vi "pharmaBot_v0.019.vi"() -> ()   [LabVIEW 2015]
uses:
  controls/user_message_v6.ctl
  pipette cleaning/pressure box/cleaning_soft/controls/arduino_pressure_setting.ctl
  <vilib>/vision/NI_Vision_Development_Module.lvlib
  <vilib>/vision/Image Controls.llb/IMAQ Image.ctl
  multiBot/patcherBot/AxMultiClampMsg.dll
  <vilib>/Platform/NI_3dgraph.lvlib
  controls/cam_type-v02.ctl
  controls/cam_info.ctl
  machine_vision/controls/transform_cluster_actuator.ctl
  <vilib>/Analysis/NI_AALBLAS.lvlib
  <vilib>/Analysis/BLAS.llb/dnrm2 - Vector 2-Norm (DBL).vi
  multipatch/controls/multipatch_individual_controls_v5.ctl
  multipatch/controls/images_controls.ctl
  machine_vision/controls/approach_type.ctl
  controls/scope_motion.ctl
  <vilib>/ptbypt/NI_PtbyPt.lvlib
  pipette cleaning/pressure box/cleaning_soft/controls/scientifica_commands.ctl
  multipatch/controls/multipatch_common_controls_v4.ctl
  controls/Load and Save Controls_LV2009.llb/RWC_Actions.ctl
  controls/memtest_def.ctl
  pipette cleaning/pressure box/cleaning_soft/controls/actuator_type.ctl
  pipette cleaning/pressure box/cleaning_soft/controls/actuator_cluster.ctl
  pipette cleaning/pressure box/cleaning_soft/controls/pressure_box_type.ctl
  pipette cleaning/pressure box/cleaning_soft/controls/pressure_box_control.ctl
  machine_vision/coordinate model vis/transform_properties_actuators.ctl
  controls/NH_method.ctl
  controls/dual_patch_controls.ctl
  wc_protocol_v1.003 Folder/whole_cell_protocol/Controls/cell_stats-v02.ctl
  multipatch/controls/Control 7b.ctl
  controls/notSureControl-v01.ctl
panel:
  in  "misc indiv":T1
  in  "Save Resistance":bool
  out "Saved Pipette Resistance":dbl caption="MOhms" format="%#_3g"
  out "allMainVIcontrols":refnum<vi>[](array[refnum])
  out "cells selected":i32
  in  "unpatched+reserved 2":i32[](array[numeric])
  out "cells left":i32
  out "ValidationOutputCluster":T2(array[cluster])=[{"daq_ao 2"="Dev1/ao1", "Duration (s)"=10.0, "Sample Freq (Hz)"=20000.0, "Phase"=-36.0, "Duty Cycle"=10.0, "Jump Filter Freq (Hz)"=30.0, "Number of Replicates"=1}, {"daq_ao 2"="", "Duration (s)"=0.0, "Sample Freq (Hz)"=0.0, "Phase"=0.0, "Duty Cycle"=0.0, "Jump Filter Freq (Hz)"=0.0, "Number of Replicates"=0}, {"daq_ao 2"="Dev1/ao1", "Duration (s)"=10.0, "Sample Freq (Hz)"=20000.0, "Phase"=-36.0, "Duty Cycle"=10.0, "Jump Filter Freq (Hz)"=30.0, "Number of Replicates"=1}, {"daq_ao 2"="Dev1/ao1", "Duration (s)"=10.0, "Sample Freq (Hz)"=20000.0, "Phase"=-36.0, "Duty Cycle"=10.0, "Jump Filter Freq (Hz)"=30.0, "Number of Replicates"=1}, {"daq_ao 2"="Dev1/ao1", "Duration (s)"=10.0, "Sample Freq (Hz)"=20000.0, "Phase"=-36.0, "Duty Cycle"=10.0, "Jump Filter Freq (Hz)"=30.0, "Number of Replicates"=1}, {"daq_ao 2"="", "Duration (s)"=0.0, "Sample Freq (Hz)"=0.0, "Phase"=0.0, "Duty Cycle"=0.0, "Jump Filter Freq (Hz)"=0.0, "Number of Replicates"=0}, {"daq_ao 2"="Dev1/ao1", "Duration (s)"=10.0, "Sample Freq (Hz)"=20000.0, "Phase"=-36.0, "Duty Cycle"=10.0, "Jump Filter Freq (Hz)"=30.0, "Number of Replicates"=1}, {"daq_ao 2"="Dev1/ao1", "Duration (s)"=10.0, "Sample Freq (Hz)"=20000.0, "Phase"=-36.0, "Duty Cycle"=10.0, "Jump Filter Freq (Hz)"=30.0, "Number of Replicates"=1}]
  out "ValidationPos2":T3(array[ring])=[enum."Experiment Safe Position", enum."Experiment Safe Position", enum."Jumper Position A", enum."Jumper Position A", enum."Experiment Safe Position", enum."Experiment Safe Position", enum."Jumper Position A", enum."Jumper Position A"]
  out "ValidationPos1":T3(array[ring])=[enum."Jumper Position B-A", enum."Jumper Position B-A", enum."Jumper Position B", enum."Jumper Position B", enum."Jumper Position B-A", enum."Jumper Position B-A", enum."Jumper Position B", enum."Jumper Position B"]
  out "ValidationResults":waveform(dbl)[][](array[waveform])=[[{"t0"=timestamp(3645556158.623614 s since 1904-01-01), "dt"=4.999999999999997e-05, "Y"=array[200000 elements], "attributes"=variant("NI_ChannelName"=variant(string "AI-jump"), "NI_UnitDescription"=variant(string "Volts"))}], [{"t0"=timestamp(3645556158.623614 s since 1904-01-01), "dt"=4.999999999999997e-05, "Y"=array[200000 elements], "attributes"=variant("NI_ChannelName"=variant(string "AI-jump"), "NI_UnitDescription"=variant(string "Volts"))}], [{"t0"=timestamp(3645556177.2816796 s since 1904-01-01), "dt"=4.999999999999997e-05, "Y"=array[200000 elements], "attributes"=variant("NI_ChannelName"=variant(string "AI-jump"), "NI_UnitDescription"=variant(string "Volts"))}], [{"t0"=timestamp(3645556195.335867 s since 1904-01-01), "dt"=4.999999999999997e-05, "Y"=array[200000 elements], "attributes"=variant("NI_ChannelName"=variant(string "AI-jump"), "NI_UnitDescription"=variant(string "Volts"))}], [{"t0"=timestamp(3645557132.4115305 s since 1904-01-01), "dt"=4.999999999999997e-05, "Y"=array[200000 elements], "attributes"=variant("NI_ChannelName"=variant(string "AI-jump"), "NI_UnitDescription"=variant(string "Volts"))}], [{"t0"=timestamp(3645557132.4115305 s since 1904-01-01), "dt"=4.999999999999997e-05, "Y"=array[200000 elements], "attributes"=variant("NI_ChannelName"=variant(string "AI-jump"), "NI_UnitDescription"=variant(string "Volts"))}], [{"t0"=timestamp(3645557151.3143697 s since 1904-01-01), "dt"=4.999999999999997e-05, "Y"=array[200000 elements], "attributes"=variant("NI_ChannelName"=variant(string "AI-jump"), "NI_UnitDescription"=variant(string "Volts"))}], [{"t0"=timestamp(3645557169.842995 s since 1904-01-01), "dt"=4.999999999999997e-05, "Y"=array[200000 elements], "attributes"=variant("NI_ChannelName"=variant(string "AI-jump"), "NI_UnitDescription"=variant(string "Volts"))}]]
  in  "Vision Fix":bool
  in  "Accept Button":bool
  in  "Valve2 Go":bool
  out "V2-Changing":bool
  out "V2-State":u16
  in  "Valve2":u16(knob) scale=1.0..8.0
  in  "Valve1 Go":bool
  out "V1-Changing":bool
  out "V1-State":u16
  in  "Valve1":u16(knob) scale=1.0..8.0
  in  "Conditions":string(combo)="Control"
  in  "AnalysisProtocol":string(combo)="NMDA_jumps_v01"
  in  "PatchSettings":string(combo)="patchSettings20180928"
  in  "Passage/Age":string(combo)="P?"
  in  "CellType":string(combo)="HEK_GABA_GluN2A"
  in  "Experiment":string(combo)="testing"
  in  "Project":string(combo)="debug"
  in  "gigasealing options 2":T4={"atm wait (indices)"=10, "num samples for slope"=5, "delta suction (mbar)"=2.0, "if less than this slope, increase suction"=1.0, "else if less than this slope, maintain suction"=100.0, "else if less than this slope, decrease suction "=200.0, "max suction (mBar)"=-40.0}
  out "cell stats":T5 {"STD" format="%010.2f"; "Variance" format="%010.2f"; "Rt (MOhms)" format="%010.2f"; "tau (ms)" format="%08.2g"; "Cm (pF)" format="%08.2f"; "Ra (MOhms)" format="%010.2f"; "Rm (MOhms)" format="%010.2f"; "Ihold (pA)" format="%010.2f"}
  in  "current manip 2 pos (steps)":i32[](array[numeric])
  in  "backlash?":bool
  out "current park plane z (px)":dbl
  in  "go to safe space":bool
  in  "set park location":bool
  in  "current manip 1 pos (steps)":i32[](array[numeric])
  in  "which action on cam":T6(radio)
  in  "delete location":bool
  in  "empty list":bool
  in  "go to cell index":bool
  in  "index":i32
  out "nWC":dbl
  out "nGS":dbl
  out "nAttempts":dbl
  out "current stage pos [um]":i32[](array[numeric]) format="%.1f"
  out "Current Manipulator Position [um]":i32[](array[numeric]) format="%.1f"
  out "current stage pos (steps)":i32[](array[numeric])
  out "Manip Being Calibrated Name":string
  out "Current Manipulator Position":i32[](array[numeric])
  in  "cell tracker XY zero adjustment (pipette 2)":dbl[](array[numeric])=[0.0, 0.0, 0.0]
  in  "cell tracker XY zero adjustment (pipette 1)":dbl[](array[numeric])=[0.0, 0.0, 0.0]
  in  "no cell tracker XY zero adjustment (px) (pipette 1 and 2)":dbl[](array[numeric])=[0.0, 0.0, 0.0]
  out "next manip position":dbl[](array[numeric])
  out "next stage position":dbl[](array[numeric])
  in  "Z focus range for pipette":i32=150
  out "Pipette is in Focus?":bool
  out "Current Manip Focus Coords.":i32[](array[numeric])
  out "Stage zeroed?":bool
  in  "Stage Shift (steps)":dbl
  in  "step distance (steps) safe space":dbl=-80000.0 format="%#_13g"
  out "Patched Cell Index":dbl
  out "Patched Cell Indicies":i32[](array[numeric])
  out "unpatched+reserved":i32[](array[numeric])
  in  "Calibration Protocol":T7(tab)
  in  "Skip Calibration Button":bool
  in  "Calibration Button":bool
  in  "How Many Manipulators?":enum16{"1", "2", "3", "4"}(ring)
  in  "Seek Backwards Calibration Button":bool
  in  "Restart Calibration Button":bool
  in  "Cancel Calibration Button":bool
  out "Manip 4 Calibrated":bool
  out "Manip 3 Calibrated":bool
  out "Manip 2 Calibrated":bool
  out "Manip 1 Calibrated":bool
  in  "Calibrate:":T8(ring)
  in  "zero stage 5":bool
  in  "zero stage":bool
  in  "zero stage 4":bool
  in  "Zero Pipette 3":bool caption="Found Pipette"
  in  "Move Stage and Pipette Down":bool caption="Found Pipette"
  in  "Pipette is in Focus":bool caption="Found Pipette"
  in  "Next Stage and Pipette Z Location":dbl(slide) scale format="%#.6g"
  in  "set safe space":bool
  in  "location above baths":bool
  in  "Manip 2 Distance [mm]":dbl=5.0
  in  "Manip 2 Angle [deg]":dbl=-100.0
  in  "Manip 1 Distance [mm]":dbl=13.0
  in  "Manip 1 Angle [deg]":dbl=-90.0
  in  "cleaning bath location":bool
  in  "wash bath location":bool
  in  "zero stage 3":bool
  in  "Zero Pipette 2":bool caption="Found Pipette"
  in  "Lower Stage 300 uM":bool
  in  "Raise Stage 300 uM":bool
  in  "send Manip to Approach Line":bool=TRUE
  in  "send Manip to XY ZERO":bool
  in  "Raise Manipulator":bool
  in  "Zero Pipette 1":bool caption="Found Pipette"
  in  "zero stage 2":bool
  in  "Zero Pipette 4":bool caption="Found Pipette"
  in  "zero stage 6":bool
  in  "go to zero":bool
  in  "Which Manip Jumper Position?":T9(ring)
  in  "Manip Jump":bool
  out "Wave Rise Time":dbl format="%#10.3g"
  out "Wave Fall Time":dbl format="%#10.3g"
  in  "Jumper Filter Freq (Hz)":dbl=30.0 min=0.0001 max=1000.0 step=0.1
  in  "go to jumper position":bool
  in  "Which Jumper Position to Set?":T9(ring)
  in  "Jump Polarity":bool
  out "Jump Rise Time":dbl format="%#10.3g"
  out "jumptestMonitor":waveform(dbl)(graph) caption="Memtest"
  out "memtestJumperMonitor":waveform(dbl)(graph) caption="Memtest"
  in  "Jump Trigger":bool
  out "Jump o-C Good?":bool
  out "Jump C-o Good?":bool
  out "Jump C-B Good?":bool
  out "Jump B-C Good?":bool
  out "Jump B-A Good?":bool
  out "Jump A-B Good?":bool
  out "Jump A-o Good?":bool
  out "Jump o-A Good?":bool
  in  "Choose Position":bool
  out "Jump Pos o-C":bool
  out "Jump Pos C-o":bool
  out "Jump Pos C-B":bool
  out "Jump Pos B-C":bool
  out "Jump Pos B-A":bool
  out "Jump Pos A-B":bool
  out "Jump Pos A-o":bool
  out "Jump Pos o-A":bool
  out "Pos C":bool
  out "Pos B":bool
  out "Pos A":bool
  out "Experiment Safe":bool
  out "Jumper Safe":bool
  out "Jump Fall Time":dbl format="%#10.3g"
  in  "save locations 2":bool
  in  "Load Cells to Queue Button":bool
  in  "Redo Calibration Button":bool
  in  "Add More Cells Button":bool
  in  "User OK":bool
  out "current cell image":T10(plugin-control)
  in  "MZ Dn":bool
  in  "MZ Up":bool
  in  "MX Up":bool
  in  "MX Dn":bool
  in  "MY Dn":bool
  in  "Manipulator Button Step Size (um)":dbl=100.0 min=0.0 step=0.1
  in  "MY Up":bool
  in  "SZ Dn":bool
  in  "SZ Up":bool
  in  "SX Up":bool
  in  "SX Dn":bool
  in  "SY Dn":bool
  in  "Stage Button Step Size (um)":dbl=100.0 min=0.0 step=0.1
  in  "SY Up":bool
  in  "Previous Patched Cell":bool
  in  "Next Patched Cell":bool
  out "Patched Cell Value":dbl
  in  "Add this cell index into queue":bool
  in  "pipette template threshold":dbl=0.6
  in  "solver_name":string="PF+RWTV-DF(ADMM)"
  in  "solver_kappa":dbl=5.0
  in  "solver_gamma":dbl=0.0003
  in  "psf_sigma":dbl=0.5
  in  "shear_angle":dbl=120.0
  in  "template_window":dbl=160.0
  in  "cell length (px)":i32=160
  out "pipette_corr_pwr":dbl
  out "pipette_tracking_quality":dbl
  out "cell_tracking_quality":dbl
  out "deconvolution output":T10(plugin-control)
  in  "P2 state":T11=enum."Setting defaults..."
  in  "P1 state":T11=enum."Setting defaults..."
  in  "current cell 2":i32
  in  "pipette 2 I (pA)":dbl(knob) min=-1000.0 max=1000.0 step=10.0 scale=-1000.0..1000.0 scale format="%#_3g"
  in  "demo pipette 2 R (MOhms)":dbl(knob)=1.0 min=1.0 max=2000.0 step=0.05 scale=2.0..2000.0
  in  "Tab Control":T12(tab)
  in  "load Settings":bool
  in  "Valve2 Connected":bool=TRUE
  in  "Valve1 Connected":bool=TRUE
  in  "Robotic Break-In?":bool=TRUE
  in  "Human in Situ":bool=TRUE
  in  "daq_ao 2":tag="Dev1/ao1"
  in  "Experimental VI To Run":string(combo)="pharmaBotExp"
  in  "daq_do 1":tag="Dev1/port1/line0:7"
  in  "Sampling Freq (Hz)":T13=20000
  in  "NH wait time (ms)":u32=1000
  in  "simultaneous WC":bool
  out "Saving to... 2":path
  in  "vertical z dist (vertical rel only)  (px)":dbl=-20000.0
  in  "HEK/slice options":enum16{"slice", "HEK"}(ring)=enum."HEK"
  in  "load HEK/slice params":bool
  in  "cell tracker":bool
  in  "skip gigasealing":bool
  in  "skip to successful breakin\n or Cell Attached Protocol":bool
  out "multiclamp on":bool
  in  "test multiclamp":bool
  out "GS timeout (adjusted)":i32=250
  in  "Data log location":path=path "C:/multiBot/data"
  in  "daq_ai":tag="Dev1/ai0"
  in  "daq_ao":tag="Dev1/ao0"
  out "Saving to... 1":path
  in  "multiclamp control?":bool=TRUE
  in  "pressure box 1":T14={"Pressure box COM"="COM4", "pressure box type"=enum."ProportionAir", "High pos pressure (mBar)"=200.0, "Low pos pressure (mBar)"=50.0, "Vacuum pressure (mBar)"=-40.0, "calibration"=enum."mightenRig"}
  in  "demo clean":bool
  in  "skip hunting":bool
  in  "skip to unsuccessful breakin":bool
  in  "demo daq?":bool
  in  "corrective pipette move":bool
  in  "Neuron Detection Threshold (MOhms)":dbl=0.1
  in  "subtract from distToDescend (steps)":i32
  in  "max hunt distance (um)":dbl=45.0
  in  "GS timeout (s)":i32=200
  in  "retract distance (um)":dbl=100.0
  out "max steps to take":i32
  in  "Extra threshold (MOhms)":dbl=0.2
  in  "Pipette broken threshold (MOhms)":dbl=-5.0
  in  "go to wash bath loc":bool
  in  "go to cleaning bath loc":bool
  in  "go to loc above baths":bool
  in  "save locations":bool
  in  "holding V (mV)":dbl=-60.0
  in  "clampex control?":bool
  in  "initial positioning":T16=enum."vertical rel"
  out "distToDescend (steps)":i32
  in  "gross descent pressure (mBar)":dbl=30.0 format="%#_13g"
  in  "NH step size (steps)":i32=10
  in  "hunt pressure (mBar)":dbl=20.0 format="%#_13g"
  in  "above dist (approach above only) (steps)":i32=-150
  in  "corrective stage move":bool
  in  "stage reservation options":T17(ring)=enum."unreserve after cell found"
  in  "cleaning tab":enum32{"manip 1", "manip 2"}(tab)
  out "loc above baths 1":i32[](array[numeric])
  out "cleaning bath loc 1":i32[](array[numeric])
  out "wash bath loc 1":i32[](array[numeric])
  out "loc above baths 2":i32[](array[numeric])
  out "cleaning bath loc 2":i32[](array[numeric])
  out "wash bath loc 2":i32[](array[numeric])
  out "GS timeout (adjusted) 2":i32=250
  in  "manip 1 on":bool=TRUE
  in  "manip 2 on":bool
  in  "NH method":T18
  out "pipette motion":T19=enum."slow_dualPatch"
  in  "Select cells based on proximity (multi patch)":bool
  in  "daq_do 2":tag="Dev1/port0/line0:7"
  out "config file":path=path "C:/multiBot/patcherBot/autoWCconfigs/autoWC_config_neuron-v07.ini"
  in  "Validate":bool
  in  "Terminate Experiment":bool
  in  "+100 mbar":bool
  in  "+20 mbar":bool
  in  "0 mbar":bool
  in  "-200 mbar":bool
  in  "+40 mV":bool
  in  "0 mV":bool
  in  "-60 mV":bool
  in  "Human Control Done":bool
  in  "In Process Calibration?":T20
  out "Break-In Counter":i32
  out "Ra 2":dbl format="%#_13g"
  out "Ra 1":dbl format="%#10.3g"
  out "successful breakin 2":bool
  out "wash bath 2 detected":bool
  out "clean bath 2 detected":bool
  out "wash bath 1 detected":bool
  out "clean bath 1 detected":bool
  out "NEURON HUNTING MONITOR":cluster{dbl[], dbl[]}(graph) caption="XY Graph"
  out "GIGASEALING MONITOR":cluster{i32[], dbl[]}(graph) caption="XY Graph"
  out "tip found 1":bool
  in  "pipette 1 broken - abort!":bool
  out "GS extended 1":bool
  out "cell found 1":bool
  in  "stage idle?":bool=TRUE
  out "NEURON HUNTING MONITOR 2":cluster{dbl[], dbl[]}(graph) caption="XY Graph"
  out "GIGASEALING MONITOR 2":cluster{i32[], dbl[]}(graph) caption="XY Graph"
  out "memtest 1":waveform(dbl)(graph)={"t0"=timestamp(3654278249.6712327 s since 1904-01-01), "dt"=4.999999999999997e-05, "Y"=array[2000 elements], "attributes"=variant("NI_ChannelName"=variant(string "Dev1/ai0"), "NI_UnitDescription"=variant(string "Volts"))} caption="Memtest"
  out "Iholding 1":dbl caption="pA" format="             %0.2f"
  out "Iholding 2":dbl caption="pA" format="%0.2f"
  out "Vholding (mV) 2":dbl
  out "Vholding (mV) 1":dbl
  out "unpatched cell indices":i32[](array[numeric])
  out "GS extended 2":bool
  in  "pipette 2 broken - abort!":bool
  out "tip found 2":bool
  out "cell found 2":bool
  in  "trial data saved":bool
  in  "trial data saved 2":bool
  in  "Command pressure (mBar) 1":dbl(slide)=-345.0 min=-700.0 max=700.0 step=0.1 scale=-700.0..700.0
  in  "Command pressure (mBar) 2":dbl(slide)=-345.0 min=-700.0 max=700.0 step=0.1 scale=-700.0..700.0
  out "initialized":bool
  in  "go to dual WC":bool
  out "successful breakin 1":bool
  out "Cm 2":dbl format="%#_13g"
  out "Cm 1":dbl format="%#10.2g"
  in  "State to advance to after Human Control":T11=enum."Gigaseal Established..."
  out "Waveform Graph":T21(graph)
  in  "cell diameter (px)":i32=100
  in  "crosshair?":bool=TRUE
  out "screen tip location (px)":i32[](array[numeric])
  out "cells (image px)":dbl[][](array[numeric])
  out "current cell locations (px)":dbl[][](array[numeric])
  in  "load 10 points":bool
  in  "Adjust exposure (ms)":dbl=0.15
  in  "camera type":T22=enum."optiMOS"
  out "cam size":i32[](array[numeric])
  out "screen tip location (px) 2":i32[](array[numeric])
  in  "Range":cluster{"Minimum":sgl, "Maximum":sgl}={"Minimum"=0.0, "Maximum"=17000.0} {"Maximum" format="%.2f"; "Minimum" format="%.2f"}
  out "cell found?":bool
  in  "cell autofocus":bool
  out "found pipette 2":T10(plugin-control)
  out "pipette mask 2":T10(plugin-control)
  out "pipette 2 template":T10(plugin-control)
  in  "pipette 2 mask":path=path "C:/multiBot/ComputerSpecificSettingsAndDefaults/pipette masks/pipette2_mask7_u8b.bmp"
  in  "temp pipette 2 template location":path=path "C:/multiBot/ComputerSpecificSettingsAndDefaults/pipette masks/temp_pipette_4_template_u16.png"
  in  "manip 2 position":T23={"width x"=314.0, "height y"=187.0, "x offset"=286.0, "y offset"=102.0}
  out "saved cell image":T10(plugin-control)
  in  "cell images":T10[](array[typedef])
  in  "cell image size (px)":i32=400
  in  "pipette 1 mask":path=path "C:/multiBot/ComputerSpecificSettingsAndDefaults/pipette masks/pipette2_mask7_u8.bmp"
  out "pipette 1 template":T10(plugin-control)
  out "pipette 1 mask":T10(plugin-control)
  in  "pipette match score":sgl=500.0
  in  "manip 1 position":T23={"width x"=314.0, "height y"=187.0, "x offset"=200.0, "y offset"=90.0}
  in  "cell match score":sgl=500.0
  in  "temp pipette 1 template location":path=path "C:/multiBot/ComputerSpecificSettingsAndDefaults/pipette masks/temp_pipette_4_template_u16.bmp"
  out "found pipette 1":T10(plugin-control)
  in  "pipette autofocus":bool
  in  "which manipulator to autofocus":T8(ring)
  out "tip found?":bool
  out "pipette score":sgl
  out "cell score":sgl
  in  "check Validation?":bool
  out "Validation Rise Time":dbl format="%#10.3g"
  out "Validation Fall Time":dbl format="%#10.3g"
  out "ValResult":waveform(dbl)[](graph)=[{"t0"=timestamp(3645557132.4115305 s since 1904-01-01), "dt"=4.999999999999997e-05, "Y"=array[200000 elements], "attributes"=variant("NI_ChannelName"=variant(string "AI-jump"), "NI_UnitDescription"=variant(string "Volts"))}] caption="Memtest"
  in  "Which Validation Phase?":u16=1
  out "Position o-C Jump Good?":bool
  out "Position C-o Jump Good?":bool
  out "Position C-B Jump Good?":bool
  out "Position B-C Jump Good?":bool
  out "Position B-A Jump Good?":bool
  out "Position A-B Jump Good?":bool
  out "Position A-o Jump Good?":bool
  out "Position o-A Jump Good?":bool
  out "Jumper Position o-C Set":bool
  out "Jumper Position C-o Set":bool
  out "Jumper Position C-B Set":bool
  out "Jumper Position B-C Set":bool
  out "Jumper Position B-A Set":bool
  out "Jumper Position A-B Set":bool
  out "Jumper Position A-o Set":bool
  out "Jumper Position o-A Set":bool
  out "Jumper Position C Set":bool
  out "Jumper Position B Set":bool
  out "Jumper Position A Set":bool
  out "Experiment Safe Position Set":bool
  out "Jumper Safe Position Set":bool
  out "Jumper Position o-C":dbl[](array[numeric])
  out "Jumper Position C-o":dbl[](array[numeric])
  out "Jumper Position C-B":dbl[](array[numeric])
  out "Jumper Position B-C":dbl[](array[numeric])
  out "Jumper Position B-A":dbl[](array[numeric])
  out "Jumper Position A-B":dbl[](array[numeric])
  out "Jumper Position A-o":dbl[](array[numeric])
  out "Jumper Position o-A":dbl[](array[numeric])
  out "Jumper Position C":dbl[](array[numeric])
  out "Jumper Position B":dbl[](array[numeric])
  out "Jumper Position A":dbl[](array[numeric])
  out "Experiment Safe Position":dbl[](array[numeric])
  out "Jumper Safe Position":dbl[](array[numeric])
  in  "coordinate model":T24(tab)
  in  "stage->cam":T25={"theta (deg)"=0.0, "X sc factor (px/step)"=0.638, "Y sc factor (px/step)"=0.638, "zero loc (x,y,z)"=[0.0, 0.0], "flip y?"=TRUE, "flip x?"=FALSE, "gamma (deg)"=25.0, "flip z?"=TRUE, "Z sc factor (px/step)"=4.8, "actuator"={"Actuator COM"="COM6", "Actuator type"=enum."Scientifica"}, "safe space (steps)"=[-69533, 0, -29190]} {"Y sc factor (px/step)" format="%#_13g"; "X sc factor (px/step)" format="%#_13g"; "theta (deg)" format="%#_13g"}
  in  "park plane z (px)":dbl
  in  "manip1->cam":T25={"theta (deg)"=0.684, "X sc factor (px/step)"=0.638, "Y sc factor (px/step)"=0.638, "zero loc (x,y,z)"=[736.8657671125733, 651.6653127226411, 63.39399999999995], "flip y?"=FALSE, "flip x?"=TRUE, "gamma (deg)"=44.0, "flip z?"=TRUE, "Z sc factor (px/step)"=36.18, "actuator"={"Actuator COM"="COM5", "Actuator type"=enum."Scientifica"}, "safe space (steps)"=[-57520, 0, -55600]} {"Y sc factor (px/step)" format="%#_13g"; "X sc factor (px/step)" format="%#_13g"; "theta (deg)" format="%#_13g"}
  in  "manip2->cam":T25={"theta (deg)"=172.0, "X sc factor (px/step)"=1.093, "Y sc factor (px/step)"=1.093, "zero loc (x,y,z)"=[640.0, 512.0, 0.0], "flip y?"=FALSE, "flip x?"=FALSE, "gamma (deg)"=25.0, "flip z?"=FALSE, "Z sc factor (px/step)"=1.093, "actuator"={"Actuator COM"="COM7", "Actuator type"=enum."Sutter"}, "safe space (steps)"=[-75437, 0, -36327]} {"Y sc factor (px/step)" format="%#_13g"; "X sc factor (px/step)" format="%#_13g"; "theta (deg)" format="%#_13g"}
  in  "current manip 3 pos (steps)":i32[](array[numeric])
  in  "manip3->cam":T25={"theta (deg)"=5.62, "X sc factor (px/step)"=0.61, "Y sc factor (px/step)"=0.61, "zero loc (x,y,z)"=[0.0, 0.0], "flip y?"=FALSE, "flip x?"=FALSE, "gamma (deg)"=25.0, "flip z?"=FALSE, "Z sc factor (px/step)"=0.61, "actuator"={"Actuator COM"="COM3", "Actuator type"=enum."Off"}, "safe space (steps)"=[-69533, 0, -29190]} {"Y sc factor (px/step)" format="%#_13g"; "X sc factor (px/step)" format="%#_13g"; "theta (deg)" format="%#_13g"}
  in  "manip4->cam":T25={"theta (deg)"=0.0, "X sc factor (px/step)"=0.61, "Y sc factor (px/step)"=0.61, "zero loc (x,y,z)"=[0.0, 0.0], "flip y?"=FALSE, "flip x?"=FALSE, "gamma (deg)"=25.0, "flip z?"=FALSE, "Z sc factor (px/step)"=0.61, "actuator"={"Actuator COM"="COM3", "Actuator type"=enum."Off"}, "safe space (steps)"=[-69533, 0, -29190]} {"Y sc factor (px/step)" format="%#_13g"; "X sc factor (px/step)" format="%#_13g"; "theta (deg)" format="%#_13g"}
  in  "current manip 4 pos (steps)":i32[](array[numeric])
  out "current pipette locations (px)":dbl[][](array[numeric])
  out "current stage location (px)":dbl[](array[numeric])
  in  "send UUX":bool
  in  "UUX":string="6.4"
  in  "send UUY":bool
  in  "send UUZ":bool
  in  "UUZ":string="6.4"
  in  "UUY":string="6.4"
  out "ValPos1":T9(ring)
  out "ValPos2":T9(ring)
  in  "breakin counter 2":i32
  in  "gigasealing options":T4={"atm wait (indices)"=10, "num samples for slope"=5, "delta suction (mbar)"=2.0, "if less than this slope, increase suction"=1.0, "else if less than this slope, maintain suction"=100.0, "else if less than this slope, decrease suction "=200.0, "max suction (mBar)"=-60.0}
  in  "GS timeout (s) slice":i32=180
  out "start GS time 1":i32
  in  "NH R":dbl[](array[numeric])
  in  "GS R":dbl[](array[numeric])
  in  "depth":dbl[](array[numeric])
  in  "time":i32[](array[numeric])
  in  "vhold applied?":bool
  in  "vhold applied? 2":bool
  out "start GS time 2":i32
  in  "time 2":i32[](array[numeric])
  in  "depth 2":dbl[](array[numeric])
  in  "NH R 2":dbl[](array[numeric])
  in  "GS R 2":dbl[](array[numeric])
  in  "breakin counter 1":i32
  in  "MAX Break In Pressure (mbar)":dbl=-200.0
  in  "hunt pressure (mBar) slice":dbl=20.0 format="%#_13g"
  in  "holding V (mV) slice":dbl=-60.0
  in  "Extra threshold (MOhms) slice":dbl=0.5
  in  "Neuron Detection Threshold (MOhms) slice":dbl=0.02
  in  "Pipette broken threshold (MOhms) slice":dbl=-5.0
  in  "max hunt distance (um) slice":dbl=35.0
  in  "d(above cell) (steps) (used to be 10) slice":i32=10
  in  "NH step size (steps) slice":i32=10
  in  "NH method slice":T18=enum."three-stepANDfixedCutOff"
  in  "Neuron Detection Threshold (MOhms) slice HEK":dbl=0.02
  in  "Extra threshold (MOhms) slice HEK":dbl=0.5
  in  "holding V (mV) slice HEK":dbl=-60.0
  in  "hunt pressure (mBar) slice HEK":dbl=20.0 format="%#_13g"
  in  "NH method slice HEK":T18=enum."three-stepANDfixedCutOff"
  in  "NH step size (steps) slice HEK":i32=10
  in  "d(above cell) (steps) (used to be 10) slice HEK":i32=250
  in  "max hunt distance (um) slice HEK":dbl=35.0
  in  "Pipette broken threshold (MOhms) slice HEK":dbl=-0.5
  in  "approach above cell (steps) HEK":i32=-150
  in  "approach above cell (steps) slice":i32=-150
  in  "GS timeout (s) HEK":i32=180
  in  "vertical z dist (vertical rel only) HEK":dbl=-10000.0
  in  "gigaseal control tab":enum32{"HEK", "slice"}(tab)
  in  "gigasealing options HEK":T4={"atm wait (indices)"=10, "num samples for slope"=5, "delta suction (mbar)"=5.0, "if less than this slope, increase suction"=10.0, "else if less than this slope, maintain suction"=100.0, "else if less than this slope, decrease suction "=200.0, "max suction (mBar)"=-60.0}
  in  "gigasealing options slice":T4={"atm wait (indices)"=10, "num samples for slope"=5, "delta suction (mbar)"=2.0, "if less than this slope, increase suction"=1.0, "else if less than this slope, maintain suction"=100.0, "else if less than this slope, decrease suction "=200.0, "max suction (mBar)"=-60.0}
  in  "NH wait time (ms) slice":u32=1000
  in  "NH wait time (ms) HEK":u32=1000
  in  "pre-clean":bool
  in  "load wash":bool
  in  "load clean":bool
  in  "Cleaning step (time [s], value [mBar]) actual":dbl[][](array[numeric])=[[5.0, -345.0], [1.0, -345.0], [1.0, 1000.0], [1.0, -345.0], [1.0, 1000.0], [1.0, -345.0], [1.0, 1000.0], [1.0, -345.0], [1.0, 1000.0], [1.0, -345.0], [1.0, 1000.0], [5.0, 1000.0]]
  out "cleaning status":string
  in  "Wash step (time [s], value [mBar]) actual":dbl[][](array[numeric])=[[3.0, -345.0], [10.0, 1000.0]]
  out "avg peak height 2":dbl
  out "avg peak height 1":dbl
  out "cleaning status 2":string
  out "mock location array":dbl[][](array[numeric])
  in  "MATLAB clearvars":bool
  in  "pipette 2 cell tracker rectangle":i32[](array[numeric])=[10, 65, 110, 115]
  out "pipette 2 mask for cell tracker":T10(plugin-control)
  out "cell tracker init error out":errorcluster
  out "centroid_px":dbl[](array[numeric])
  out "exit tracker success":bool
  in  "solver_beta":dbl
  out "init tracker success":bool
  out "cell tracking box (px)":i32[](array[numeric])
  out "cell track error out":errorcluster
  in  "tracking":bool
  out "cell mask ROI":T28 {"Contours"."Type" items=["No Selection", "Point", "Line", "Rectangle", "Oval", "Polygon", "Freehand Region", "Annulus", "Unused2", "Unused3", "Broken Line", "Freehand Line", "Rotated Rectangle"]}
  out "run tracker success":bool
  in  "debug_mode":bool
  out "pipette_px_onscreen":dbl[](array[numeric])
  in  "pipette 1 cell tracker rectangle":i32[](array[numeric])=[214, 40, 314, 90]
  out "pipette 1 mask for cell tracker":T10(plugin-control)
  out "cell tracking box (px) 2":i32[](array[numeric])
  out "tip select error":errorcluster
  out "pipette corrMask":T10(plugin-control)
  in  "Power Spectrum inputs":T29={"Samples to Read"=10000, "Rate (Hz)"=20000.0, "Amplitude (mV/pA)"=10.0, "Offset (mV/pA)"=0.0, "Frequency (Hz)"=10.0, "duty cycle (%)"=50.0, "phase"=-90.0} {"phase" format="%.2p"; "duty cycle (%)" format="%0.2f"}
  out "mclamp cluster":T30
  out "Multiclamp Handle":u32=722860
  in  "channels to initialize":T31(array[ring])=[enum."manipulator 1", enum."manipulator 2"]
  in  "Memtest inputs":T29={"Samples to Read"=2000, "Rate (Hz)"=20000.0, "Amplitude (mV/pA)"=10.0, "Offset (mV/pA)"=0.0, "Frequency (Hz)"=10.0, "duty cycle (%)"=50.0, "phase"=90.0} {"phase" format="%.2p"; "duty cycle (%)" format="%0.2f"}
  out "pipette offset (mV) 2":dbl
  out "pipette offset (mV)":dbl
  in  "initial memtest inputs":T29={"Samples to Read"=2000, "Rate (Hz)"=20000.0, "Amplitude (mV/pA)"=10.0, "Offset (mV/pA)"=0.0, "Frequency (Hz)"=10.0, "duty cycle (%)"=50.0, "phase"=-90.0} {"phase" format="%.2p"; "duty cycle (%)" format="%0.2f"}
  in  "check Power Specturm":bool
  in  "dual WC keep going":bool=TRUE
  in  "dual patch cluster":T32={"sampling rate (Hz)"=20000.0, "total duration (s)"=5.0, "stim amplitude (pA)"=2000.0, "time between stims (s)"=3.0, "delta t (s)"=0.01, "pulse width (s)"=0.002, "# repetitions"=3.0, "number of pulses"=10, "before stim (s)"=1.0}
  out "state list manip 2":string[](array[string])
  out "state times 2":dbl[](array[numeric])
  out "previous time in":timestamp
  out "state list manip 1":string[](array[string])
  out "state times 1":dbl[](array[numeric])
  out "stop always":bool
  in  "stop memtest":bool
  out "Power Spectrum":dbl[](graph)
  out "Power Spectrum Current":waveform(dbl)[](graph)
  in  "3D Graph":refnum<k7>(container)
  out "camera":T33(graph)
  out "cell centroid graph":cluster{dbl[], dbl[]}(graph)
  out "manip distance (steps)":dbl
  out "stage distance (steps)":dbl
  out "measured manip 1 difference (steps)":i32[](array[numeric])
  out "measured stage difference (steps)":i32[](array[numeric])
  in  "zero manip measurement":bool
  in  "zero stage measurement":bool
  out "Distances":sgl[](array[numeric]) format="%.4f"
  out "pipette centroid graph":cluster{dbl[], dbl[]}(graph)
  out "cell centroid array":dbl[][](array[numeric])
  out "pipette centroid array":dbl[][](array[numeric])
  in  "stop":bool
  out "P2":dbl caption="MOhms" format="%#_3g"
  out "P1":dbl caption="MOhms" format="%#_3g"
  out "individual controls manip 2":T34
  out "positions":T35
  out "transforms":T36
  out "common controls":T37
  out "individual controls manip 1":T34
  out "measured stage zero (steps)":i32[](array[numeric])
  out "measured manip 1 zero (steps)":i32[](array[numeric])
  out "orig image":T10
  out "cam info out":T38={"camera type"=enum."Qcam", "cam handle"=0, "data handle"=0, "cam size"=[]}
  in  "pipette 1 I (pA)":dbl(knob) min=-1000.0 max=1000.0 step=10.0 scale=-1000.0..1000.0 scale format="%#_3g"
  in  "demo pipette 1 R (MOhms)":dbl(knob)=1.0 min=1.0 max=2000.0 step=0.05 scale=2.0..2000.0
  out "Slice view":T10(plugin-control)
  in  "current cell 1":i32
  out "save path":path
  # "Debugging Only"
  # "cells Selected"
  # "GS"
  # "WC"
  # "Att"
  # "cells left"
  # "Stage [um]:"
  # "Manip Pos [um]:"
  # "Stage:"
  # "Calibration UI"
  # "In order to run the program, please ensure that the system is calibrated prior to running any experiments. On this page, please specify the number of manipulators in this setup if you plan to calibrate the system."
  # "Select Manipulator to Calibrate"
  # "Select the manipulator that you whish to calibrate here. The LEDs indicate which manipulators have been calibrated since running the program."
  # "Set the 0 Position for the Stage"
  # "(don't adjust other locations)"
  # "(update other locations)"
  # "Find the Pipette Under the Microscope"
  # "New Pipette (don't adjust other locations)\nor Error Adjustment after large movements"
  # "(don't adjust other locations)"
  # "CELLS"
  # "Set Safe Space"
  # "Move the pipette to a location that is safe for the pipette to return to. This is usually placed at a location away from the workspace but along the line of approach."
  # "Set the Safe Pipette Height ABOVE the Bath"
  # "Move the pipette to a position that is located ABOVE the baths. Placing the pipette a couple of mm above the fluid height is good enough."
  # "Set the Location of the CLEANING Bath"
  # "Place the tip of the pipette in the cleaning solution."
  # "Set the Location of the WASHING Bath"
  # "Place the pipette in the wash bath"
  # "Make Sure Pipette Returns to '0'"
  # "Check again to make sure that manipulator returns to the correct location in the @mutiBot camera window. If there is any error, you can reset the manipulator's '0' location now."
  # "Pipette Adjustment (update other locations)\nie altering the zero location after error check"
  # "(update other locations)"
  # "Pipette Adjustment (update other locations)\nie altering the zero location after error check"
  # "New Pipette (don't adjust other locations)\nor Error Adjustment after large movements"
  # "(update other locations)"
  # "(don't adjust other locations)"
  # "Position Set?"
  # "Low"
  # "High"
  # "Jumper Position Legend"